vi "20200213_CHF.vi"() -> ()   [LabVIEW 2017] (continued)
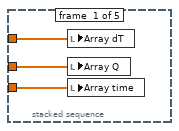
[diagram p2: hidden frame]
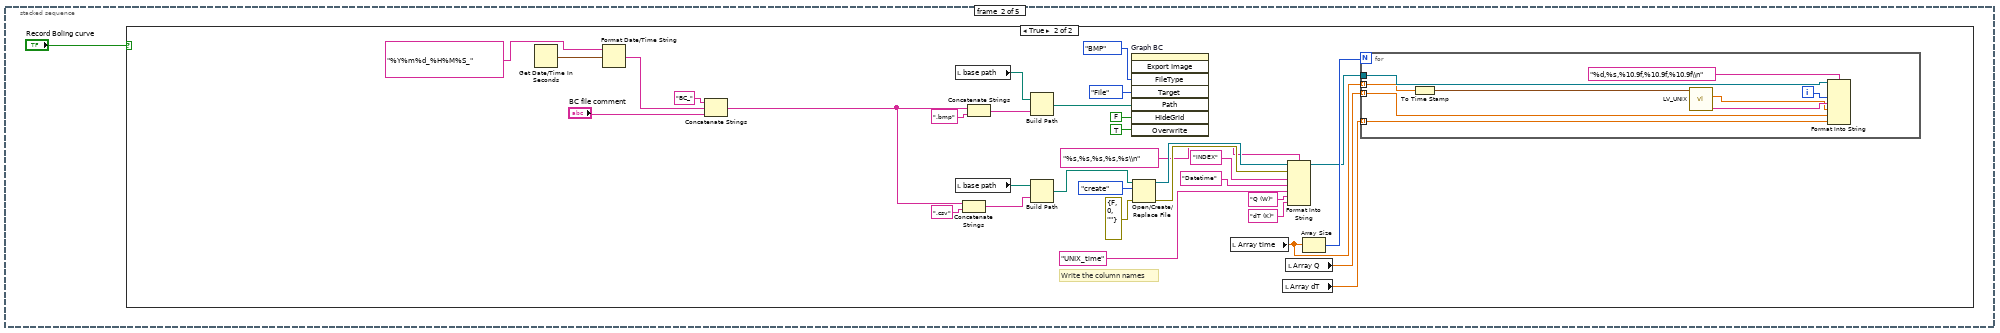
[diagram p3: hidden frame]
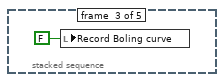
[diagram p5: hidden frame]
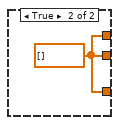
[diagram p6: hidden frame]
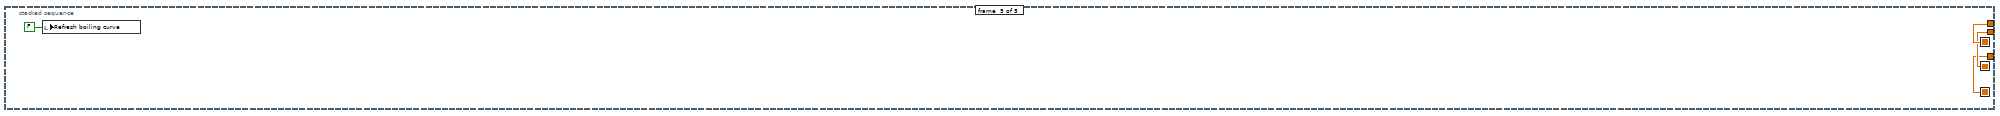
[diagram p7: hidden frame]
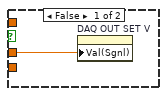
[diagram p9: hidden frame]
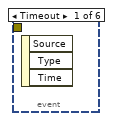
[diagram p10: hidden frame]
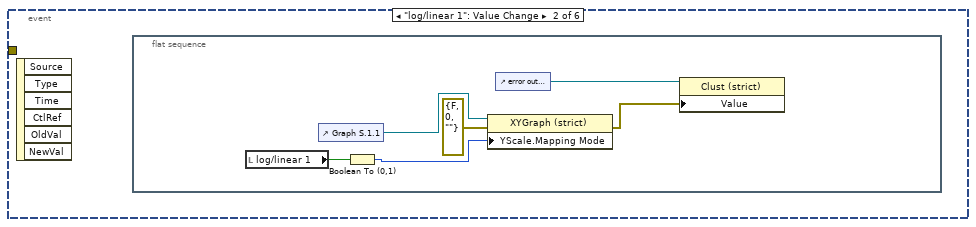
[diagram p11: hidden frame]
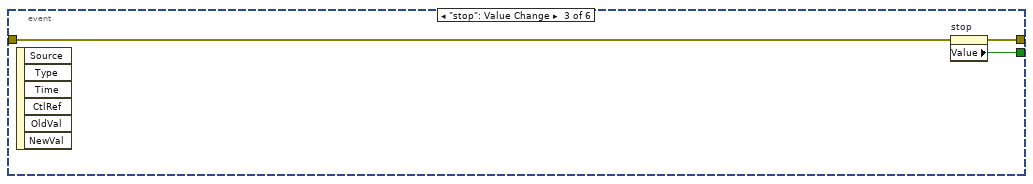
[diagram p12: hidden frame]
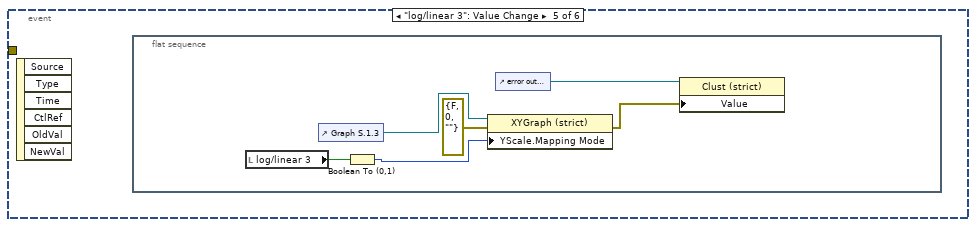
[diagram p13: hidden frame]
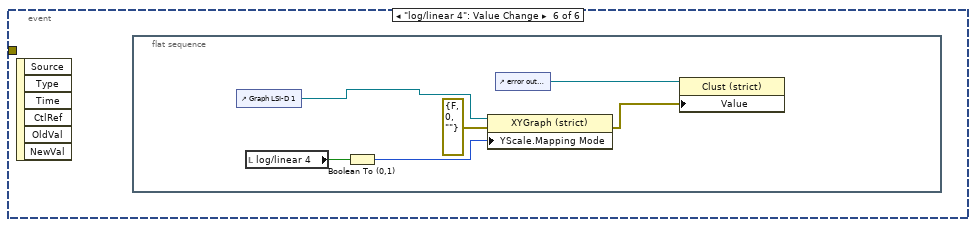
[diagram p14: hidden frame]
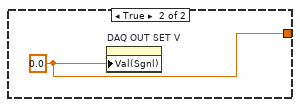
[diagram p15: hidden frame]
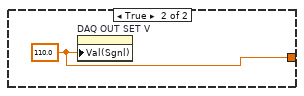
[diagram p16: hidden frame]
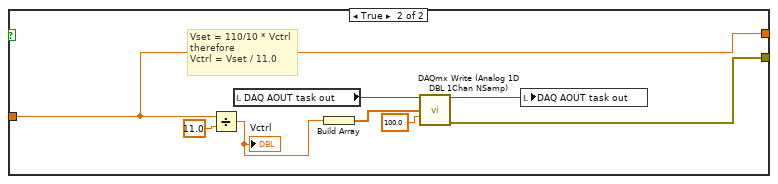
[diagram p17: hidden frame]
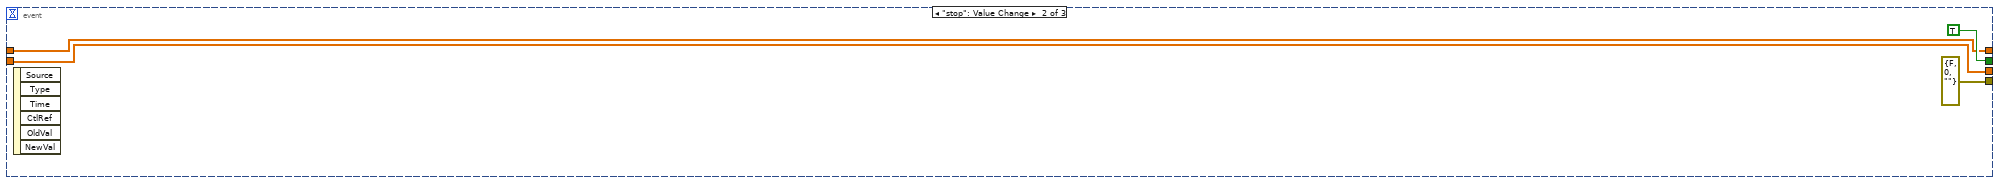
[diagram p18: hidden frame]
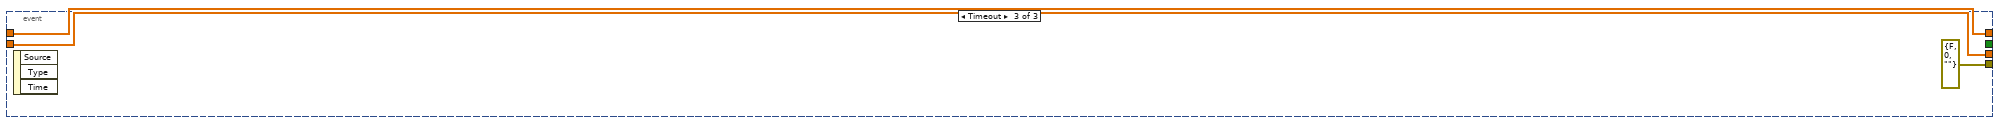
[diagram p19: hidden frame]
            n145 = Divide(x=w507, y=w499) -> (x/y=w502:dbl)
            n146 = call "scaling_calculator.vi"("x1"=1.0, "y1"=0.0 ("x1"), "x"=w502, "x2"=5.0 ("x1"), "y2"=200000.0 ("x1")) -> ("y"=w500:dbl)  [unwired: 2 in]
          }
          frame #8 {
            # "8"
            # "AI17 absolute pressure"
            n147 = Add Array Elements(numeric array=w509) -> (sum=w516:dbl)
            n148 = Divide(x=w516, y=w508) -> (x/y=w511:dbl)
            n149 = call "scaling_calculator.vi"("x1"=1.0, "y1"=0.0 ("x1"), "x"=w511, "x2"=5.0 ("x1"), "y2"=200000.0 ("x1")) -> ("y"=w510:dbl)  [unwired: 2 in]
          }
          frame #9 {
            # "9"
            # "AIN18 baratron front"
            n150 = Add Array Elements(numeric array=w520) -> (sum=w522:dbl)
            n151 = Divide(x=w522, y=w517) -> (x/y=w519:dbl)
            n152 = case shown="False" TRUE {
              tunnel: [w524 w525] -> w521
              tunnel: w519 -> [w523 w526]
              frame False {
                n153 = call "scaling_calculator_baratron.vi"("x"=w523) -> ("y (Pa)"=w524:dbl)  [unwired: 5 in, 1 out]
              }
              frame True {
                n154 = call "baratron_conv_analog.vi"("V_ana (V)"=w526) -> ("y (Pa)"=w525:dbl)  [unwired: 10 in]
              }
            }
          }
          frame #10 {
            # "10"
            # "AIN 19 baratron buffer 1\n--> in this version, changed to voltage readout of the heater"
            n155 = Add Array Elements(numeric array=w531) -> (sum=w532:dbl)
            n156 = Divide(x=w532, y=w530) -> (x/y=w529:dbl)
            n157 = Divide(x=w529, y="Rv/(Rv+Ro)") -> (x/y=w527:dbl)
          }
          frame #11 {
            # "11"
            # "AIN20 baratron buffer 2\n-->AIN23  Volage over 10Ohm resistor is converted to current"
            n158 = Add Array Elements(numeric array=w537) -> (sum=w538:dbl)
            n159 = Divide(x=w538, y=w536) -> (x/y=w535:dbl)
            n160 = Divide(x=w535, y="Ri (Ohm)") -> (x/y=w534:dbl)
          }
          frame #12 {
            # "AIN21 leak detector exp"
            n161 = Add Array Elements(numeric array=w546) -> (sum=w547:dbl)
            n162 = Divide(x=w547, y=w539) -> (x/y=w545:dbl)
            n163 = Round To Nearest(number=w545) -> (nearest integer value=w544:dbl)
            n164 = Add(x=w544, y=2.0) -> (x+y=w542:dbl)
            n165 = Multiply(x=w542, y=-1.0) -> (x*y=w540:dbl)
          }
          frame #13 {
            # "AIN21 leak detector mantissa"
            n166 = Add Array Elements(numeric array=w550) -> (sum=w551:dbl)
            n167 = Divide(x=w551, y=w548) -> (x/y=w549:dbl)
          }
        }
        n168 = Power Of 10(x=w270) -> (10^x=w268:dbl)
        n169 = Multiply(x=w269, y=w268) -> (x*y=w267:dbl)
        n170 = Build Array(w343, w341, w340, w337, w336, w335, w333, w318, w285, w286, w248, w251, w270, w269, w267) -> (w254:dbl[])
        "DAQ AIN CONV" <- w254
        n171 = local write "OUT S.1 1"(w254) -> ()
        n172 = local write "OUT S.1.2"(w254) -> ()
        n173 = Build Array (concatenate)(w344, w254) -> (w317:dbl[][])
        n174 = Index Array(array=w317, index (col) #1=0 ("disabled index (col)"), index (col) #2=1 ("disabled index (col)"), index (col) #3=2 ("disabled index (col)"), index (col) #4=3 ("disabled index (col)"), index (col) #5=4 ("index (col)"), index (col) #6=5 ("index (col)"), index (col) #7=6 ("index (col)"), index (col) #8=7 ("index (col)"), index (col) #9=8 ("index (col)"), index (col) #10=9 ("index (col)"), index (col) #11=10 ("index (col)"), index (col) #12=11 ("index (col)"), index (col) #13=12 ("index (col)"), index (col) #14=13 ("index (col)"), index (col) #15=14 ("index (col)")) -> (element #1=w355:dbl[], element #2=w353:dbl[], element #3=w351:dbl[], element #4=w349:dbl[], element #5=w346:dbl[], element #6=w345:dbl[], element #7=w279:dbl[], element #8=w278:dbl[], element #9=w308:dbl[], element #10=w291:dbl[], element #11=w289:dbl[], element #12=w283:dbl[], element #13=w262:dbl[], element #14=w261:dbl[], element #15=w260:dbl[])  [unwired: 15 in]
        n175 = Bundle(w263, w355) -> (w312:cluster{dbl[], dbl[]})  [unwired: 1 in]
        n176 = Bundle(w263, w353) -> (w311:cluster{dbl[], dbl[]})  [unwired: 1 in]
        n177 = Bundle(w263, w351) -> (w307:cluster{dbl[], dbl[]})  [unwired: 1 in]
        n178 = Bundle(w263, w349) -> (w306:cluster{dbl[], dbl[]})  [unwired: 1 in]
        n179 = Bundle(w263, w346) -> (w305:cluster{dbl[], dbl[]})  [unwired: 1 in]
        n180 = Bundle(w263, w345) -> (w304:cluster{dbl[], dbl[]})  [unwired: 1 in]
        n181 = Bundle(w263, w279) -> (w303:cluster{dbl[], dbl[]})  [unwired: 1 in]
        n182 = Bundle(w263, w278) -> (w302:cluster{dbl[], dbl[]})  [unwired: 1 in]
        n183 = Bundle(w263, w308) -> (w301:cluster{dbl[], dbl[]})  [unwired: 1 in]
        n184 = Bundle(w263, w291) -> (w290:cluster{dbl[], dbl[]})  [unwired: 1 in]
        n185 = Bundle(w263, w289) -> (w288:cluster{dbl[], dbl[]})  [unwired: 1 in]
        n186 = Bundle(w263, w283) -> (w282:cluster{dbl[], dbl[]})  [unwired: 1 in]
        n187 = Bundle(w263, w262) -> (w259:cluster{dbl[], dbl[]})  [unwired: 1 in]
        n188 = Bundle(w263, w261) -> (w258:cluster{dbl[], dbl[]})  [unwired: 1 in]
        n189 = Bundle(w263, w260) -> (w257:cluster{dbl[], dbl[]})  [unwired: 1 in]
        n190 = Build Array(w312, w311, w307, w306, w305, w304, w303, w302, w301, w290, w288, w282, w259, w258, w257) -> (w300:cluster{dbl[], dbl[]}[])
        n191 = stacked-sequence {
          tunnel: w300 -> [w405 w417 w429]
          frame #0 {
            n192 = local read "DAQ AIN CH indic."() -> (w402:string[])
            n193 = Array Size(array=w402) -> (size(s)=w404:i32)
            n194 = for {
              N: w404 -> [_]
              tunnel: [w409] -> w403
              tunnel: w402 -> [w408] mode=indexing
              i -> [w411]
              n195 = control-ref of="Graph S.1.1"() -> (w407:refnum<vi>)
              n196 = property class="XYGraph (strict)"(reference=w407, error in=errorcluster {"status"=FALSE, "code"=0, "source"=""} ("error in (no error)"), "Active Plot"=w411, "Plot.Plot Name"=w408) -> (error out=w409:errorcluster)  [unwired: 1 out]
            }
            n197 = control-ref of="Graph S.1.1"() -> (w401:refnum<vi>)
            n198 = property class="XYGraph (strict)"(reference=w401, error in=w403, "Val(Sgnl)"=w405) -> (error out=w406:errorcluster)  [unwired: 1 out]
            n199 = control-ref of="error out (decoration)"() -> (w400:refnum<vi>)
            n200 = property class="Clust (strict)"(reference=w400, "Value"=w406) -> ()  [unwired: 1 in, 2 out]
          }
          frame #1 {
            n201 = local read "DAQ AIN CH indic."() -> (w414:string[])
            n202 = Array Size(array=w414) -> (size(s)=w416:i32)
            n203 = for {
              N: w416 -> [_]
              tunnel: [w421] -> w415
              tunnel: w414 -> [w420] mode=indexing
              i -> [w423]
              n204 = control-ref of="Graph S.1.2"() -> (w419:refnum<vi>)
              n205 = property class="XYGraph (strict)"(reference=w419, error in=errorcluster {"status"=FALSE, "code"=0, "source"=""} ("error in (no error)"), "Active Plot"=w423, "Plot.Plot Name"=w420) -> (error out=w421:errorcluster)  [unwired: 1 out]
            }
            n206 = control-ref of="Graph S.1.2"() -> (w412:refnum<vi>)
            n207 = property class="XYGraph (strict)"(reference=w412, error in=w415, "Val(Sgnl)"=w417) -> (error out=w418:errorcluster)  [unwired: 1 out]
            n208 = control-ref of="error out (decoration)"() -> (w413:refnum<vi>)
            n209 = property class="Clust (strict)"(reference=w413, "Value"=w418) -> ()  [unwired: 1 in, 2 out]
          }
          frame #2 {
            n210 = local read "DAQ AIN CH indic."() -> (w426:string[])
            n211 = control-ref of="Graph S.1.3"() -> (w424:refnum<vi>)
            n212 = Array Size(array=w426) -> (size(s)=w428:i32)
            n213 = for {
              N: w428 -> [_]
              tunnel: [w433] -> w427
              tunnel: w426 -> [w432] mode=indexing
              tunnel: w424 -> [w431]
              i -> [w435]
              n214 = property class="XYGraph (strict)"(reference=w431, error in=errorcluster {"status"=FALSE, "code"=0, "source"=""} ("error in (no error)"), "Active Plot"=w435, "Plot.Plot Name"=w432) -> (error out=w433:errorcluster)  [unwired: 1 out]
            }
            n215 = property class="XYGraph (strict)"(reference=w424, error in=w427, "Val(Sgnl)"=w429) -> (error out=w430:errorcluster)  [unwired: 1 out]
            n216 = control-ref of="error out (decoration)"() -> (w425:refnum<vi>)
            n217 = property class="Clust (strict)"(reference=w425, "Value"=w430) -> ()  [unwired: 1 in, 2 out]
          }
        }
      }
    }
    n218 = flat-sequence {
      tunnel: w234 -> [w565]
      tunnel: w238 -> [w597]
      tunnel: [w595] -> w235
      tunnel: [w566] -> w230
      tunnel: w228 -> [w567]
      tunnel: w227 -> [w561]
      tunnel: w226 -> [w560]
      tunnel: w225 -> [w557]
      tunnel: w224 -> [w556]
      tunnel: [w674] -> w236
      tunnel: w235 -> [w674]
      tunnel: [w673] -> w231
      tunnel: w230 -> [w673]
      tunnel: [w691] -> w237
      tunnel: w236 -> [w691]
      tunnel: [w686] -> w229
      tunnel: w231 -> [w686]
      frame #0 {
        n219 = call "Data Sensor.vi"("VISA resource name"=w561, "error in (no error)"=w560) -> ("Input 1"=w606:dbl, "Input 2"=w605:dbl, "Input 3"=w604:dbl, "VISA resource name out"=w598:refnum<visa-resource-name>, "Input 4"=w596:dbl, "Input 5"=w603:dbl, "Input 6"=w602:dbl, "Input 8"=w600:dbl, "Input 7"=w601:dbl, "error out"=w599:errorcluster)  [unwired: 4 in]
        n220 = control-ref of="error out (LSI)"() -> (w558:refnum<vi>)
        n221 = case shown="False" FALSE {
          tunnel: w567 -> [w607 w616]
          tunnel: [w607 w615] -> w566
          tunnel: w565 -> [_ w614]
          tunnel: w557 -> [_ w611]
          tunnel: w556 -> [_ w610]
          frame False {
          }
          frame True {
            n222 = call "Data Sensor.vi"("VISA resource name"=w610, "error in (no error)"=w611) -> ("Input 1"=w651:dbl, "Input 2"=w650:dbl, "Input 3"=w649:dbl, "VISA resource name out"=w653:refnum<visa-resource-name>, "Input 4"=w648:dbl, "Input 5"=w647:dbl, "Input 6"=w646:dbl, "Input 8"=w644:dbl, "Input 7"=w645:dbl, "error out"=w652:errorcluster)  [unwired: 4 in]
            n223 = control-ref of="error out (LSI)"() -> (w613:refnum<vi>)
            n224 = Build Array(w651, w650, w649, w648, w647, w646, w645, w644) -> (w608:dbl[])
            "LSI-U out" <- w608
            "LSI-U out 1" <- w608
            n225 = call "Close.vi"("VISA resource name"=w653, "error in (no error)"=w652) -> ("error out"=w612:errorcluster)  [unwired: 13 in]
            n226 = property class="Clust (strict)"(reference=w613, "Value"=w612) -> ()  [unwired: 1 in, 2 out]
            n227 = Build Array (concatenate)(w616, w608) -> (w615:dbl[][])
            n228 = Index Array(array=w615, index (col) #1=0 ("disabled index (col)"), index (col) #2=1 ("index (col)"), index (col) #3=2 ("index (col)"), index (col) #4=3 ("index (col)"), index (col) #5=4 ("index (col)"), index (col) #6=5 ("index (col)"), index (col) #7=6 ("index (col)"), index (col) #8=7 ("index (col)"), index (col) #9=8 ("index (col)")) -> (element #1=w618:dbl[], element #2=w627:dbl[], element #3=w628:dbl[], element #4=w629:dbl[], element #5=w630:dbl[], element #6=w631:dbl[], element #7=w632:dbl[], element #8=w633:dbl[], element #9=w634:dbl[])  [unwired: 9 in]
            n229 = Bundle(w614, w618) -> (w635:cluster{dbl[], dbl[]})  [unwired: 1 in]
            n230 = Bundle(w614, w627) -> (w636:cluster{dbl[], dbl[]})  [unwired: 1 in]
            n231 = Bundle(w614, w628) -> (w637:cluster{dbl[], dbl[]})  [unwired: 1 in]
            n232 = Bundle(w614, w629) -> (w638:cluster{dbl[], dbl[]})  [unwired: 1 in]
            n233 = Bundle(w614, w630) -> (w639:cluster{dbl[], dbl[]})  [unwired: 1 in]
            n234 = Bundle(w614, w631) -> (w640:cluster{dbl[], dbl[]})  [unwired: 1 in]
            n235 = Bundle(w614, w632) -> (w641:cluster{dbl[], dbl[]})  [unwired: 1 in]
            n236 = Bundle(w614, w633) -> (w642:cluster{dbl[], dbl[]})  [unwired: 1 in]
            n237 = Bundle(w614, w634) -> (w643:cluster{dbl[], dbl[]})  [unwired: 1 in]
            n238 = Build Array(w635, w636, w637, w638, w639, w640, w641, w642, w643) -> (w609:cluster{dbl[], dbl[]}[])
            n239 = local write "Graph LSI-U 1"(w609) -> ()
          }
        }
        n240 = Build Array(w606, w605, w604, w596, w603, w602, w601, w600) -> (w554:dbl[])
        "LSI-D out" <- w554
        "LSI-D out 1" <- w554
        n241 = call "Close.vi"("VISA resource name"=w598, "error in (no error)"=w599) -> ("error out"=w559:errorcluster)  [unwired: 13 in]
        n242 = property class="Clust (strict)"(reference=w558, "Value"=w559) -> ()  [unwired: 1 in, 2 out]
        n243 = Build Array (concatenate)(w597, w554) -> (w595:dbl[][])
        n244 = Index Array(array=w595, index (col) #1=0 ("disabled index (col)"), index (col) #2=1 ("index (col)"), index (col) #3=2 ("index (col)"), index (col) #4=3 ("index (col)"), index (col) #5=4 ("index (col)"), index (col) #6=5 ("index (col)"), index (col) #7=6 ("index (col)"), index (col) #8=7 ("index (col)"), index (col) #9=8 ("index (col)")) -> (element #1=w593:dbl[], element #2=w584:dbl[], element #3=w583:dbl[], element #4=w582:dbl[], element #5=w581:dbl[], element #6=w580:dbl[], element #7=w579:dbl[], element #8=w578:dbl[], element #9=w577:dbl[])  [unwired: 9 in]
        n245 = Bundle(w565, w593) -> (w576:cluster{dbl[], dbl[]})  [unwired: 1 in]
        n246 = Bundle(w565, w584) -> (w575:cluster{dbl[], dbl[]})  [unwired: 1 in]
        n247 = Bundle(w565, w583) -> (w574:cluster{dbl[], dbl[]})  [unwired: 1 in]
        n248 = Bundle(w565, w582) -> (w573:cluster{dbl[], dbl[]})  [unwired: 1 in]
        n249 = Bundle(w565, w581) -> (w572:cluster{dbl[], dbl[]})  [unwired: 1 in]
        n250 = Bundle(w565, w580) -> (w571:cluster{dbl[], dbl[]})  [unwired: 1 in]
        n251 = Bundle(w565, w579) -> (w570:cluster{dbl[], dbl[]})  [unwired: 1 in]
        n252 = Bundle(w565, w578) -> (w569:cluster{dbl[], dbl[]})  [unwired: 1 in]
        n253 = Bundle(w565, w577) -> (w568:cluster{dbl[], dbl[]})  [unwired: 1 in]
        n254 = Build Array(w576, w575, w574, w573, w572, w571, w570, w569, w568) -> (w555:cluster{dbl[], dbl[]}[])
        n255 = local write "Graph LSI-D 1"(w555) -> ()
        n256 = feedback #2() -> (w563:errorcluster)  [unwired: 1 in]
        n257 = stacked-sequence {
          tunnel: [w656 _] -> w564
          tunnel: [_ w665] -> w562
          tunnel: w563 -> [_ w664]
          frame #0 {
            n258 = local read "LSI-D CH indic."() -> (w655:string[])
            n259 = control-ref of="Graph LSI-D 1"() -> (w654:refnum<vi>)
            n260 = Array Size(array=w655) -> (size(s)=w657:i32)
            n261 = for {
              N: w657 -> [_]
              tunnel: [w660] -> w656
              tunnel: w655 -> [w659] mode=indexing
              tunnel: w654 -> [w658]
              i -> [w661]
              n262 = property class="XYGraph (strict)"(reference=w658, error in=errorcluster {"status"=FALSE, "code"=0, "source"=""} ("error in (no error)"), "Active Plot"=w661, "Plot.Plot Name"=w659) -> (error out=w660:errorcluster)  [unwired: 1 out]
            }
          }
          frame #1 {
            n263 = local read "LSI-U CH indic,"() -> (w666:string[])
            n264 = control-ref of="Graph LSI-U 1"() -> (w663:refnum<vi>)
            n265 = Array Size(array=w666) -> (size(s)=w667:i32)
            n266 = for {
              N: w667 -> [_]
              tunnel: w666 -> [w671] mode=indexing
              tunnel: [w670] -> w665
              tunnel: w664 -> [w669]
              tunnel: w663 -> [w668]
              i -> [w672]
              n267 = property class="XYGraph (strict)"(reference=w668, error in=w669, "Active Plot"=w672, "Plot.Plot Name"=w671) -> (error out=w670:errorcluster)  [unwired: 1 out]
            }
          }
        }
        n268 = feedback-in #2(w564) -> ()
        n269 = control-ref of="error out (decoration)"() -> (w553:refnum<vi>)
        n270 = property class="Clust (strict)"(reference=w553, "Value"=w562) -> ()  [unwired: 1 in, 2 out]
      }
      frame #1 {
      }
      frame #2 {
        n271 = case shown="True" FALSE {
          frame False {
          }
          frame True {
            n272 = local read "LSI-U out"() -> (w704:dbl[])
            n273 = local read "current time"() -> (w708:timestamp)
            n274 = Array To Cluster(array=w704) -> (cluster=w707:T5)
            n275 = local read "ref LSI-U"() -> (w703:refnum<file>)
            n276 = local read "Cycle #"() -> (w711:i32)
            n277 = To Double Precision Float(number=w708) -> (double precision float=w705:dbl)
            n278 = call "LV_UNIX.vi"("current time"=w708) -> ("date/time string"=w710:string, "UNIX time (s)"=w709:dbl)  [unwired: 9 in]
            n279 = Unbundle(w707) -> ("LSI-U out[0]"=w700:dbl, "LSI-U out[1]"=w701:dbl, "LSI-U out[2]"=w702:dbl, "LSI-U out[3]"=w699:dbl, "LSI-U out[4]"=w698:dbl, "LSI-U out[5]"=w697:dbl, "LSI-U out[6]"=w696:dbl, "LSI-U out[7]"=w695:dbl)  [unwired: 1 out]
            n280 = Format Into String(format string="%d,%s,%10.4f,%10.4f,%5.6f,%5.6f,%5.6f,%5.6f,%5.6f,%5.6f,%5.6f,%5.6f\\n", initial string=w703, w711, w710, w709, w705, w700, w701, w702, w699, w698, w697, w696, w695) -> ()  [unwired: 1 in, 2 out]
          }
        }
        n281 = local read "LSI-D out"() -> (w685:dbl[])
        n282 = local read "current time"() -> (w690:timestamp)
        n283 = Array To Cluster(array=w685) -> (cluster=w692:T6)
        n284 = local read "ref LSI-D"() -> (w684:refnum<file>)
        n285 = local read "Cycle #"() -> (w687:i32)
        n286 = To Double Precision Float(number=w690) -> (double precision float=w694:dbl)
        n287 = call "LV_UNIX.vi"("current time"=w690) -> ("date/time string"=w688:string, "UNIX time (s)"=w689:dbl)  [unwired: 9 in]
        n288 = Unbundle(w692) -> ("LSI-D out[0]"=w683:dbl, "LSI-D out[1]"=w682:dbl, "LSI-D out[2]"=w681:dbl, "LSI-D out[3]"=w680:dbl, "LSI-D out[4]"=w679:dbl, "LSI-D out[5]"=w678:dbl, "LSI-D out[6]"=w677:dbl, "LSI-D out[7]"=w676:dbl)  [unwired: 1 out]
        n289 = Format Into String(format string="%d,%s,%10.4f,%10.4f,%5.6f,%5.6f,%5.6f,%5.6f,%5.6f,%5.6f,%5.6f,%5.6f\\n", initial string=w684, w687, w688, w689, w694, w683, w682, w681, w680, w679, w678, w677, w676) -> ()  [unwired: 1 in, 2 out]
      }
    }
    n290 = local read "DAQ AOUT task out"() -> (w223:refnum<k21>)
    "Cycle #" <- w240
  }
  n291 = while {
    tunnel: w2 -> [w721]
    tunnel: [w721] -> w11
    shift-right: [w713] -> _
    shift-left: w5 -> [w715]
    shift-right: [w712] -> _
    shift-left: w5 -> [w714]
    i -> [w716]
    stop <- "stop" stop-if-true
    n292 = event shown="[0] \"DAQ OUT SET V\", \"DAQ OUT ON?\": Value Change" {
      selector: _ -> [_ _ _]
      dyn-events: _ -> [_ _ _]
      timeout: _ -> [_ _ _]
      tunnel: [w738 errorcluster {"status"=FALSE, "code"=0, "source"=""} ("error out") errorcluster {"status"=FALSE, "code"=0, "source"=""} ("error out")] -> w718
      tunnel: [_ TRUE _] -> _
      tunnel: w714 -> [w733 w761 w764]
      tunnel: [w731 w761 w764] -> w712
      tunnel: w715 -> [w730 w762 w765]
      tunnel: [w729 w762 w765] -> w713
      event "DAQ OUT SET V", "DAQ OUT ON?": Value Change {
        w723 = 11.0 ("y")
        # "return x only when 0<=x<=10"
        n293 = event-data() -> ()  [unwired: 1 in, 6 out]
        n294 = Get Date/Time In Seconds() -> (seconds since 1Jan1904=w728:timestamp)
        n295 = local read "V_lim_max"() -> (w726:dbl)
        n296 = local read "V_lim_min"() -> (w724:dbl)
        n297 = To Double Precision Float(number=w728) -> (double precision float=w727:dbl)
        n298 = Multiply(x=w724, y=w723) -> (x*y=w722:dbl)
        n299 = Multiply(x=w726, y=w723) -> (x*y=w725:dbl)
        n300 = Build Array (concatenate)(w730, w727) -> (w729:dbl[])
        n301 = Greater?(x="DAQ OUT SET V", y=w725) -> (0:w736:bool)
        n302 = case shown="False" w736 {
          tunnel: w722 -> [w742 _]
          tunnel: "DAQ OUT SET V" -> [w739 _]
          tunnel: [w740 w745] -> w735
          frame False {
            n303 = Less?(x=w739, y=w742) -> (x < y?=w741:bool)
            n304 = case shown="False" w741 {
              tunnel: [w743 w744] -> w740
              tunnel: w739 -> [w743 _]
              frame False {
              }
              frame True {
                w744 = 0.0 ("y")
                n305 = property on="DAQ OUT SET V" class="DigNum (strict)"("Val(Sgnl)"=w744) -> ()  [unwired: 2 in, 2 out]
              }
            }
          }
          frame True {
            w745 = 110.0 ("y")
            n306 = property on="DAQ OUT SET V" class="DigNum (strict)"("Val(Sgnl)"=w745) -> ()  [unwired: 2 in, 2 out]
          }
        }
        n307 = case shown="False" "DAQ OUT ON?" {
          tunnel: [w747 w758] -> w738
          tunnel: [w746 w753] -> w732
          tunnel: w735 -> [_ w753]
          frame False {
            w746 = 0.0 ("element")
            n308 = local read "DAQ AOUT task out"() -> (w751:refnum<k21>)
            n309 = Build Array(w746) -> (w748:dbl[])
            n310 = call <vilib>:"DAQmx Write (Analog 1D DBL 1Chan NSamp).vi"("task/channels in"=w751, "data"=w748, "timeout"=100.0) -> ("task out"=w750:refnum<k21>, "error out"=w747:errorcluster)  [unwired: 10 in, 1 out]
            n311 = local write "DAQ AOUT task out"(w750) -> ()
          }
          frame True {
            # "Vset = 110/10 * Vctrl\ntherefore \nVctrl = Vset / 11.0"
            n312 = Divide(x=w753, y=11.0) -> (x/y=w752:dbl)
            "Vctrl" <- w752
            n313 = local read "DAQ AOUT task out"() -> (w757:refnum<k21>)
            n314 = Build Array(w752) -> (w755:dbl[])
            n315 = call <vilib>:"DAQmx Write (Analog 1D DBL 1Chan NSamp).vi"("task/channels in"=w757, "data"=w755, "timeout"=100.0) -> ("task out"=w756:refnum<k21>, "error out"=w758:errorcluster)  [unwired: 10 in, 1 out]
            n316 = local write "DAQ AOUT task out"(w756) -> ()
          }
        }
        n317 = Build Array (concatenate)(w733, w732) -> (w731:dbl[])
      }
      event "stop": Value Change {
        n318 = event-data() -> ()  [unwired: 1 in, 6 out]
      }
      event Timeout {
        n319 = event-data() -> ()  [unwired: 1 in, 3 out]
      }
    }
    "error out (DAQ AOU)" <- w718
    n320 = Wait (ms)(milliseconds to wait=u32 50) -> ()  [unwired: 1 out]
    n321 = Bundle(w713, w712) -> (→"Graph V SET":cluster{dbl[], dbl[]})  [unwired: 1 in]
    "cycle # CTRL" <- w716
  }
  n322 = while {
    tunnel: w2 -> [w793]
    tunnel: [w792] -> w6
    tunnel: w1 -> [w778]
    shift-right: [w775] -> _
    shift-left: w1 -> [w767]
    shift-right: [w774] -> _
    shift-left: w1 -> [w773]
    shift-right: [w770] -> _
    shift-left: w1 -> [w769]
    i -> [w795]
    stop <- w794 stop-if-true
    n323 = Wait (ms)(milliseconds to wait="dt (ms) (>50)") -> ()  [unwired: 1 out]
    n324 = stacked-sequence {
      seq-local: [_ _ _ w847 _] -> [_ _ _ _ w855]
      seq-local: [_ _ _ w846 _] -> [_ _ _ _ w854]
      seq-local: [_ _ _ w844 _] -> [_ _ _ _ w853]
      tunnel: w767 -> [w797 _ _ _ _]
      tunnel: w773 -> [w798 _ _ _ _]
      tunnel: w769 -> [w799 _ _ _ _]
      tunnel: [_ _ _ _ w855] -> w777
      tunnel: [_ _ _ _ w854] -> w776
      tunnel: [_ _ _ _ w853] -> w768
      frame #0 {
        n325 = local write "Array dT"(w797) -> ()
        n326 = local write "Array Q"(w798) -> ()
        n327 = local write "Array time"(w799) -> ()
      }
      frame #1 {
        n328 = case shown="True" "Record Boling curve" {
          frame False {
          }
          frame True {
            # "Write the column names"
            n329 = Get Date/Time In Seconds() -> (seconds since 1Jan1904=w827:timestamp)
            n330 = Format Date/Time String(time format string (%c)="%Y%m%d_%H%M%S_", seconds (now)=w827) -> (date/time string=w829:string)  [unwired: 1 in]
            n331 = Concatenate Strings("BC_" ("string"), w829, "BC file comment") -> (w811:string)
            n332 = local read "base path"() -> (w812:path)
            n333 = local read "base path"() -> (w830:path)
            n334 = Concatenate Strings(w811, ".csv" ("string")) -> (w813:string)
            n335 = Concatenate Strings(w811, ".bmp" ("string")) -> (w809:string)
            n336 = Build Path(base path=w812, name or relative path=w809) -> (appended path=w808:path)
            n337 = Build Path(base path=w830, name or relative path=w813) -> (appended path=w831:path)
            n338 = invoke on="Graph BC" class="XYGraph (strict)" method="Export Image"("FileType"=enum32{"BMP", "EPS", "EMF", "PICT"}."BMP" ("File Type"), "Target"=enum32{"File", "Clipboard"}."File", "Path"=w808, "HideGrid"=FALSE ("Hide Grid"), "Overwrite"=TRUE ("Always Overwrite")) -> ()  [unwired: 3 in, 8 out]
            n339 = Open/Create/Replace File(file path (use dialog)=w831, error in=errorcluster {"status"=FALSE, "code"=0, "source"=""}, operation (0:open)=T2."create") -> (refnum out=w832:refnum<file>, error out=w833:errorcluster)  [unwired: 3 in, 1 out]
            n340 = local read "Array time"() -> (w803:dbl[])
            n341 = local read "Array dT"() -> (w801:dbl[])
            n342 = local read "Array Q"() -> (w802:dbl[])
            n343 = Format Into String(format string="%s,%s,%s,%s,%s\\n" ("time format string (%c)"), initial string=w832, error in=w833, "INDEX" ("input 1"), "Datetime" ("input 1"), "UNIX_time" ("input 1"), "Q (W)" ("input 4"), "dT (K)" ("input 5")) -> (resulting string=w815:refnum<file>)  [unwired: 1 out]
            n344 = Array Size(array=w803) -> (size(s)=w816:i32)
            n345 = for {
              N: w816 -> [_]
              tunnel: w815 -> [w842]
              tunnel: w803 -> [w840] mode=indexing
              tunnel: w802 -> [w835] mode=indexing
              tunnel: w801 -> [w834] mode=indexing
              i -> [w838]
              n346 = To Time Stamp(1:w840) -> (0:w839:timestamp)
              n347 = call "LV_UNIX.vi"("current time"=w839) -> ("date/time string"=w837:string, "UNIX time (s)"=w836:dbl)  [unwired: 9 in]
              n348 = Format Into String(format string="%d,%s,%10.9f,%10.9f,%10.9f\\n", initial string=w842, w838, w837, w836, w835, w834) -> ()  [unwired: 1 in, 2 out]
            }
          }
        }
      }
      frame #2 {
        n349 = local write "Record Boling curve"(FALSE ("Record Boling curve")) -> ()
      }
      frame #3 {
        n350 = case shown="False" "Refresh boiling curve" {
          tunnel: [w850 w851] -> w847
          tunnel: [w849 w851] -> w846
          tunnel: [w848 w851] -> w844
          frame False {
            n351 = local read "Array time"() -> (w848:dbl[])
            n352 = local read "Array dT"() -> (w850:dbl[])
            n353 = local read "Array Q"() -> (w849:dbl[])
          }
          frame True {
            w851 = dbl[] []
          }
        }
      }
      frame #4 {
        n354 = local write "Refresh boiling curve"(FALSE ("Boling curve \nRefresh")) -> ()
      }
    }
    n355 = flat-sequence {
      tunnel: w795 -> [_]
      frame #0 {
        n356 = case shown="True" "DAQ-O \nAUTO CTL" {
          frame False {
          }
          frame True {
            n357 = local read "DAQ OUT SET V"() -> (w857:dbl)
            n358 = local read "DAQ OUT MAX (V)"() -> (w861:dbl)
            n359 = local read "DAQ OUT MIN (V)"() -> (w860:dbl)
            n360 = Add(x="dV/cycle (V)", y=w857) -> (x+y=w858:dbl)
            n361 = In Range and Coerce(upper limit=w861, x=w858, lower limit=w860) -> (In Range?=w859:bool)  [unwired: 1 out]
            n362 = case shown="True" w859 {
              tunnel: w857 -> [_ _]
              tunnel: w858 -> [_ w864]
              tunnel: w857 -> [w863 _]
              frame False {
                n363 = property on="DAQ OUT SET V" class="DigNum (strict)"("Val(Sgnl)"=w863) -> ()  [unwired: 2 in, 2 out]
              }
              frame True {
                n364 = property on="DAQ OUT SET V" class="DigNum (strict)"("Val(Sgnl)"=w864) -> ()  [unwired: 2 in, 2 out]
              }
            }
          }
        }
      }
    }
    n365 = property on="stop" class="Bool (strict)"(error in=w793) -> (error out=w792:errorcluster, "Value"=w794:bool)  [unwired: 1 in, 1 out]
    n366 = local read "OUT S.1 1"() -> (w787:dbl[])
    n367 = local read "LSI-D out"() -> (w791:dbl[])
    n368 = Index Array(array=w787, index=10) -> (element=w782:dbl)
    "V (V)" <- w782
    n369 = Index Array(array=w787, index=11) -> (element=w781:dbl)
    "I (A)" <- w781
    n370 = Index Array(array=w791, index=1) -> (element=w785:dbl)
    "T_Cu (K)" <- w785
    n371 = Index Array(array=w791, index=0) -> (element=w784:dbl)
    "T_He (K)" <- w784
    n372 = Get Date/Time In Seconds() -> (seconds since 1Jan1904=w772:timestamp)
    n373 = Subtract(x=w785, y=w784) -> (x-y=w783:dbl)
    n374 = Multiply(x=w782, y=w781) -> (x*y=w780:dbl)
    n375 = To Double Precision Float(number=w772) -> (double precision float=w771:dbl)
    n376 = Build Array (concatenate)(w777, w783) -> (w775:dbl[])
    n377 = Build Array (concatenate)(w768, w771) -> (w770:dbl[])
    n378 = Build Array (concatenate)(w776, w780) -> (w774:dbl[])
    n379 = Bundle(w775, w774) -> (→"Graph BC":cluster{dbl[], dbl[]})  [unwired: 1 in]
    "Array dT" <- w778
    "Array Q" <- w778
    "Array time" <- w778
  }
  n380 = Merge Errors(w12, w11, w10, w6) -> (w13:errorcluster)
  n381 = call <vilib>:"DAQmx Stop Task.vi"("task/channels in"=w20, "error in"=w13) -> ("task out"=w22:refnum<k21>, "error out"=w21:errorcluster)  [unwired: 12 in]
  n382 = call <vilib>:"DAQmx Clear Task.vi"("task in"=w22, "error in"=w21) -> ("error out"=w24:errorcluster)  [unwired: 13 in]
  n383 = call <vilib>:"DAQmx Stop Task.vi"("task/channels in"=w19, "error in"=w24) -> ("task out"=w25:refnum<k21>, "error out"=w23:errorcluster)  [unwired: 12 in]
  n384 = call <vilib>:"DAQmx Clear Task.vi"("task in"=w25, "error in"=w23) -> ("error out"=w4:errorcluster)  [unwired: 13 in]
  n385 = invoke on="stop" class="Bool (strict)" method="Reinit To Default"(error in=w4) -> (error out=→"error out (end)":errorcluster)  [unwired: 2 in, 2 out]
